vi "snake client.vi"() -> ()   [LabVIEW 2015]
uses:
  <vilib>/event_ctls.llb/eventvkey.ctl
  <vilib>/picture/picture.llb/Draw True-Color Pixmap.vi
panel:
  in  "path":path
  out "score 1":i32
  out "VKey":T1
  out "score 2":i32
  out "2D Picture":picture
  out "Numeric":i32
  out "x .and. y?":bool
  out "food x":i32
  out "food y":i32
  out "x":i32
  out "y":i32
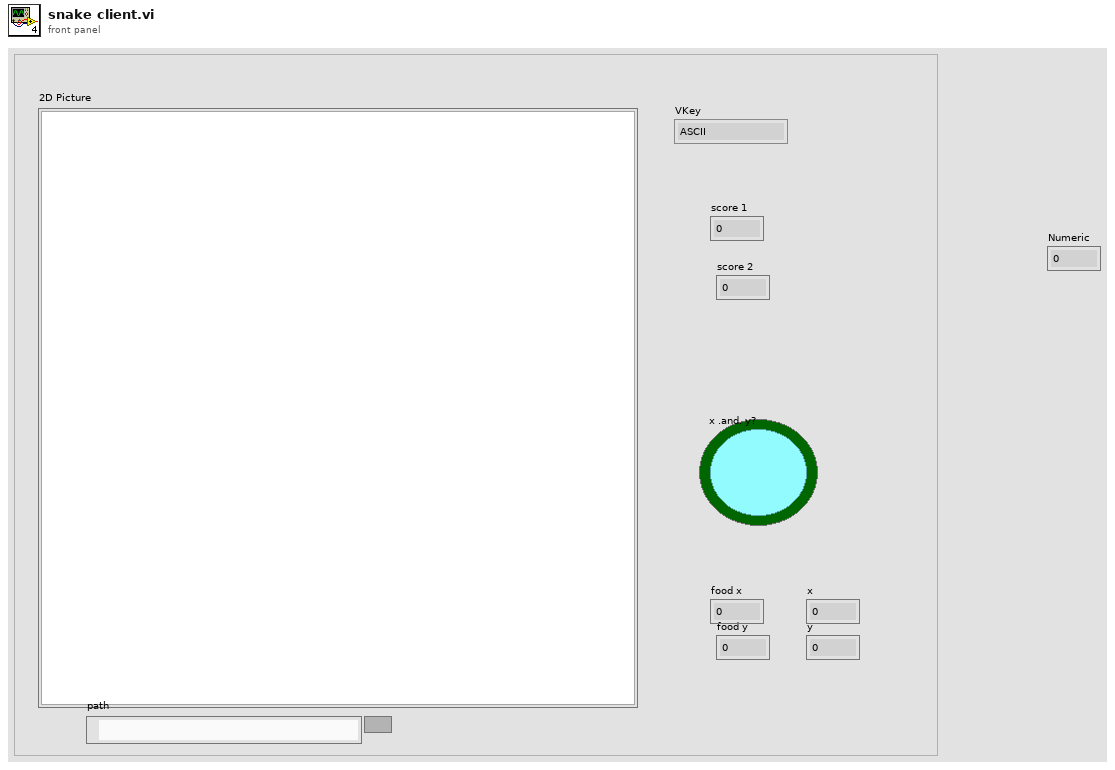
[diagram p1: front panel]
types:
  T1 = typedef "eventvkey.ctl" = enum16{"ASCII", "Enter", "Return", "Shift", "Ctrl", "Alt", "Cmd", "Opt", "Caps", "NumLock", "Clear", "Break", "Up", "Down", "Left", "Right", "Insert", "Delete", "Home", "End", "PageUp", "PageDown", "Escape", "Help", "Pause", "ScrollLock", "F1", "F2", "F3", "F4", "F5", "F6", "F7", "F8", "F9", "F10", "F11", "F12", "F13", "F14", "F15", "F16", "F17", "F18", "F19", "F20", "F21", "F22", "F23", "F24", "Play", "VolumeUp", "VolumeDown", "Mute", "Two Byte Char"}
  T2 = enum16{"Read", "Write", "ReadWrite", "BufferedRead", "BufferedReadWrite"}
  T3 = cluster{"direction":string, "snake x":i32[], "snake y":i32[]}
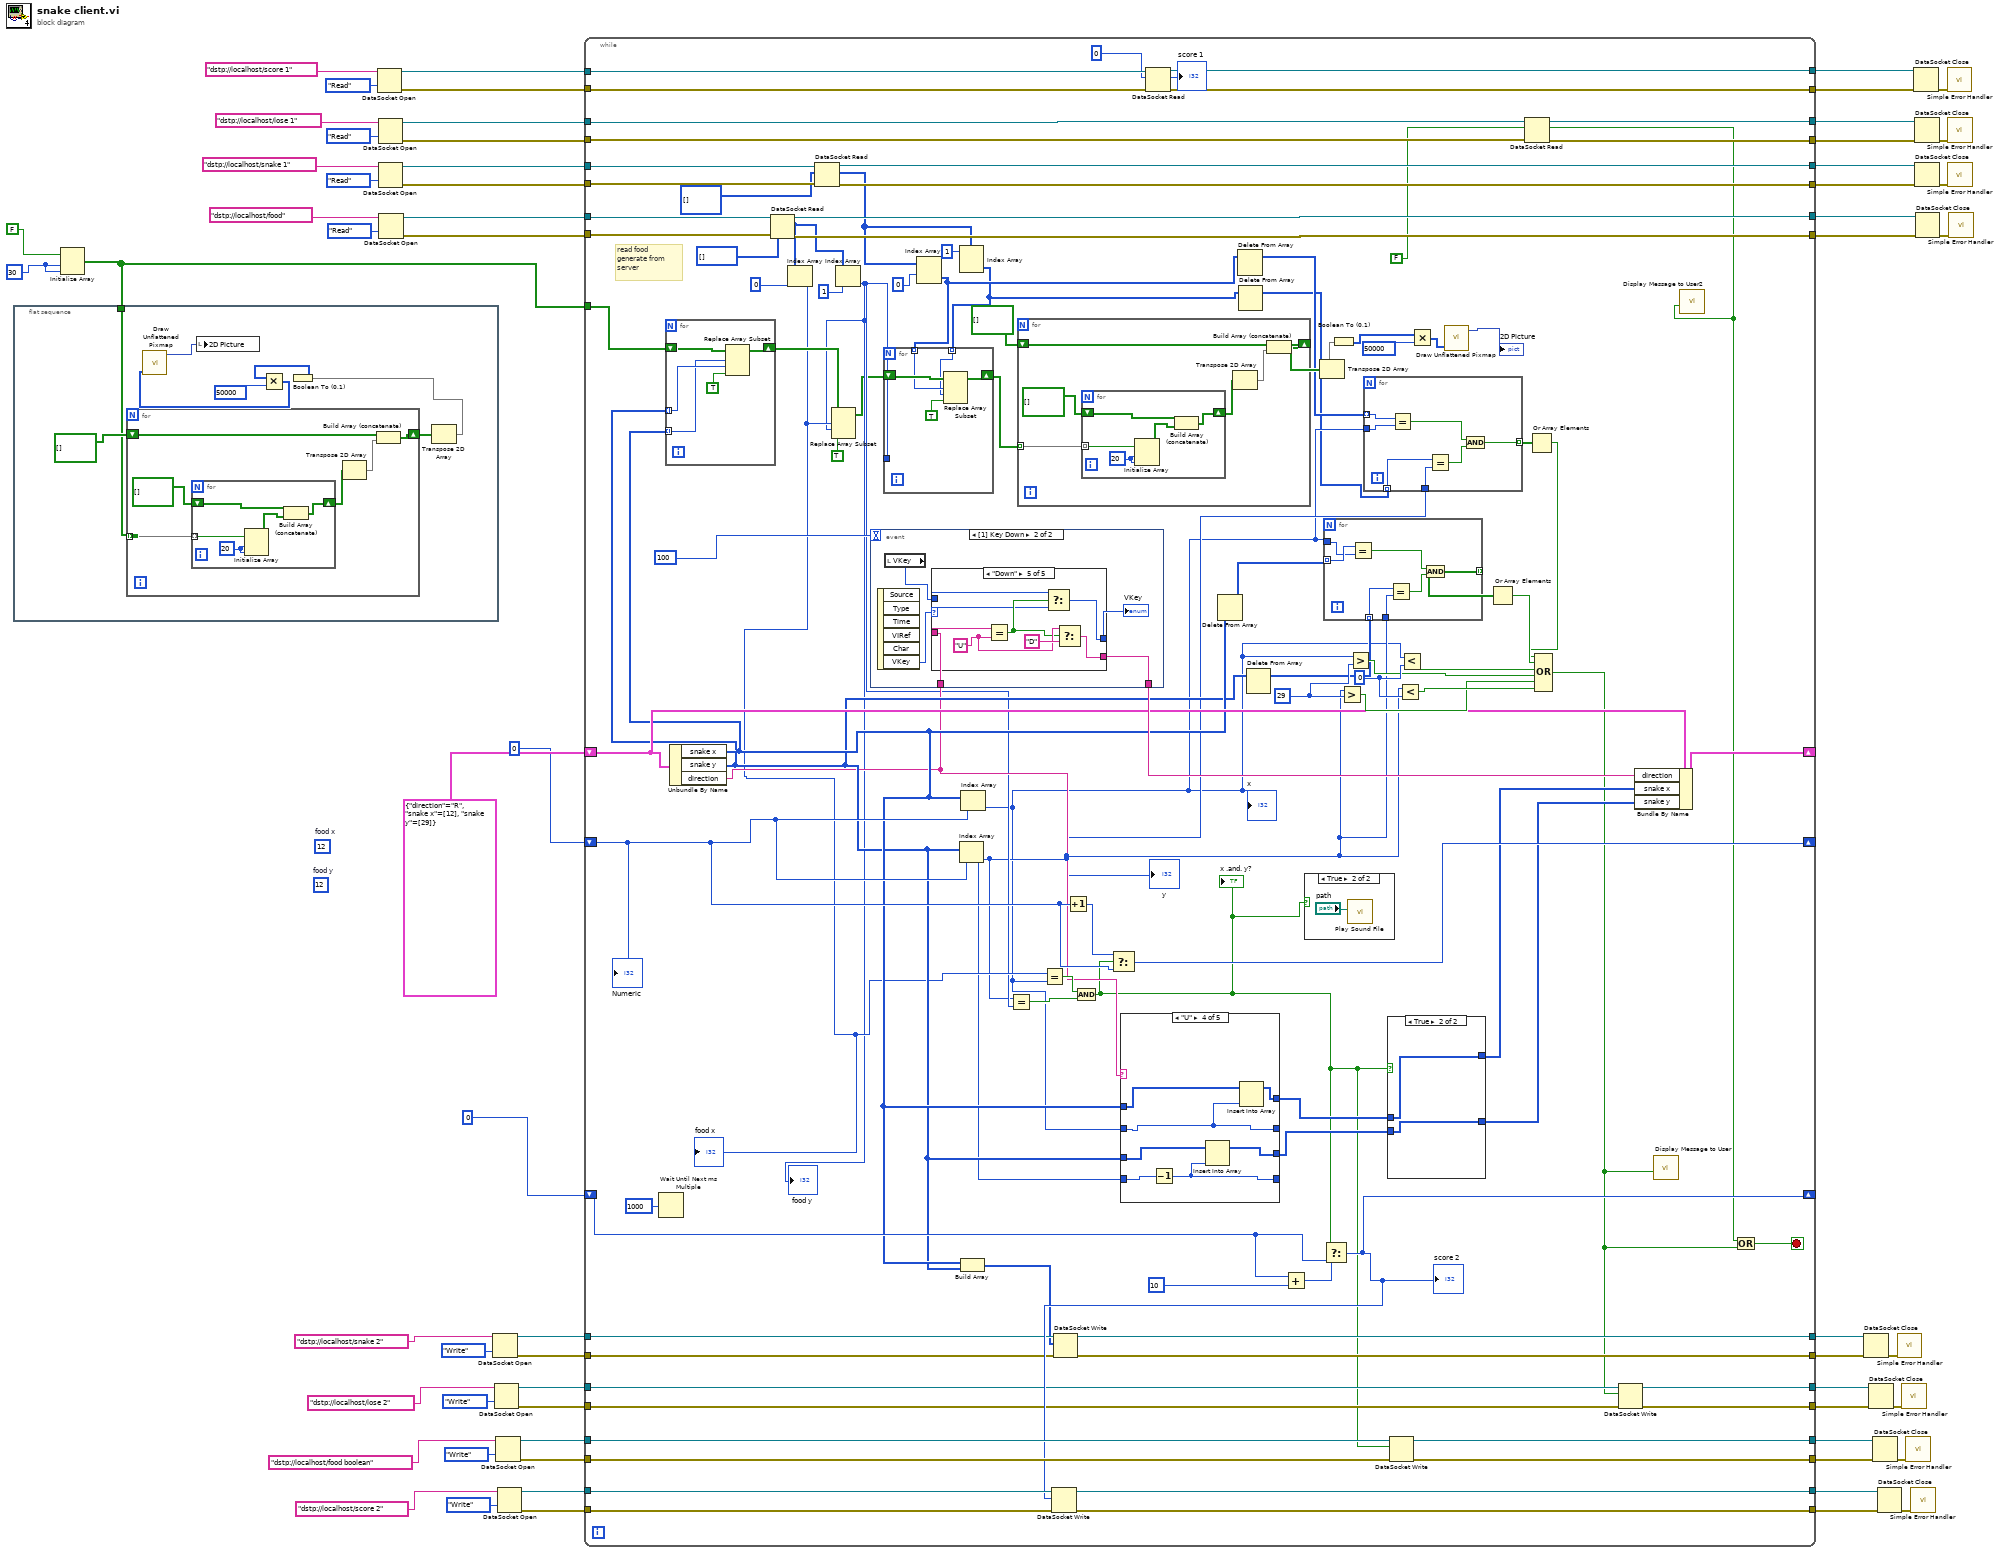
[diagram p0: block diagram]
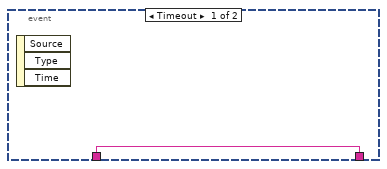
[diagram p3: hidden frame]
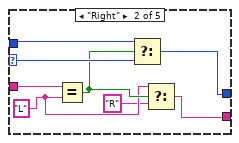
[diagram p5: hidden frame]
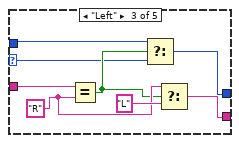
[diagram p6: hidden frame]
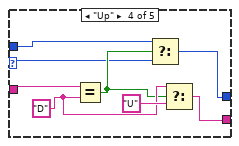
[diagram p7: hidden frame]
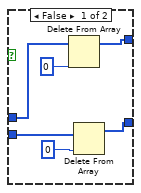
[diagram p8: hidden frame]
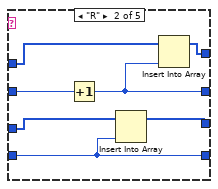
[diagram p10: hidden frame]
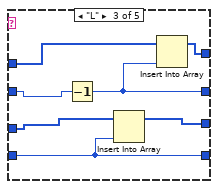
[diagram p11: hidden frame]
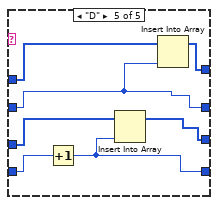
[diagram p12: hidden frame]
diagram:
  (unwired) 12  # food y
  (unwired) 12  # food x
  w59 = 30
  n1 = flat-sequence {
    tunnel: w57 -> [w63]
    frame #0 {
      n2 = for {
        tunnel: w63 -> [w76] mode=indexing
        shift-right: [w71] -> w69
        shift-left: bool[][] [] -> [w72]
        n3 = for {
          tunnel: w76 -> [w81] mode=indexing
          shift-right: [w77] -> w74
          shift-left: bool[][] [] -> [w78]
          w80 = 20
          n4 = Initialize Array(w81, w80, w80) -> (w79:bool[][])
          n5 = Build Array (concatenate)(w78, w79) -> (w77:bool[][])
        }
        n6 = Transpose 2D Array(2D array=w74) -> (transposed array=w73:bool[][])
        n7 = Build Array (concatenate)(w72, w73) -> (w71:bool[][])
      }
      n8 = Transpose 2D Array(2D array=w69) -> (transposed array=w68:bool[][])
      n9 = Boolean To (0,1)(Boolean=w68) -> (0, 1=w67:i16[][])
      n10 = Multiply(x=w67, y=50000) -> (x*y=w65:i32[][])
      n11 = call-poly <vilib>:"Draw Unflattened Pixmap.vi"("data (RGB format)"=w65) -> ("new picture"=w64:picture)  [unwired: 8 in]
      n12 = local write "2D Picture"(w64) -> ()
    }
  }
  n13 = Initialize Array(FALSE, w59, w59) -> (w57:bool[][])
  n14 = DataSocket Open(10:T2."Read" ("mode"), 11:"dstp://localhost/score 1" ("URL")) -> (0:w19:errorcluster, 3:w18:refnum<k13>)  [unwired: 2 in]
  n15 = DataSocket Open(10:T2."Read" ("mode"), 11:"dstp://localhost/lose 1" ("URL")) -> (0:w10:errorcluster, 3:w11:refnum<k13>)  [unwired: 2 in]
  n16 = DataSocket Open(10:T2."Read" ("mode"), 11:"dstp://localhost/snake 1" ("URL")) -> (0:w22:errorcluster, 3:w23:refnum<k13>)  [unwired: 2 in]
  n17 = DataSocket Open(10:T2."Read" ("mode"), 11:"dstp://localhost/food" ("URL")) -> (0:w43:errorcluster, 3:w42:refnum<k13>)  [unwired: 2 in]
  n18 = DataSocket Open(10:T2."Write" ("mode"), 11:"dstp://localhost/snake 2" ("URL")) -> (0:w34:errorcluster, 3:w33:refnum<k13>)  [unwired: 2 in]
  n19 = DataSocket Open(10:T2."Write" ("mode"), 11:"dstp://localhost/lose 2" ("URL")) -> (0:w38:errorcluster, 3:w37:refnum<k13>)  [unwired: 2 in]
  n20 = DataSocket Open(10:T2."Write" ("mode"), 11:"dstp://localhost/food boolean" ("URL")) -> (0:w55:errorcluster, 3:w56:refnum<k13>)  [unwired: 2 in]
  n21 = DataSocket Open(10:T2."Write" ("mode"), 11:"dstp://localhost/score 2" ("URL")) -> (0:w48:errorcluster, 3:w49:refnum<k13>)  [unwired: 2 in]
  n22 = while {
    shift-right: [w182] -> _
    shift-left: T3 {"direction"="R", "snake x"=[12], "snake y"=[29]} -> [w145]
    shift-right: [w178] -> _
    shift-left: 0 -> [w176]
    shift-right: [w134] -> _
    shift-left: 0 -> [w151]
    tunnel: w57 -> [w159]
    tunnel: w56 -> [w147]
    tunnel: w55 -> [w146]
    tunnel: [w144] -> w53
    tunnel: [w143] -> w52
    tunnel: w49 -> [w142]
    tunnel: w48 -> [w141]
    tunnel: [w140] -> w46
    tunnel: [w139] -> w45
    tunnel: w43 -> [w137]
    tunnel: w42 -> [w138]
    tunnel: [w136] -> w40
    tunnel: [w135] -> w39
    tunnel: w33 -> [w133]
    tunnel: w34 -> [w132]
    tunnel: w37 -> [w131]
    tunnel: w38 -> [w130]
    tunnel: [w129] -> w27
    tunnel: [w128] -> w28
    tunnel: [w127] -> w31
    tunnel: [w126] -> w32
    tunnel: w22 -> [w120]
    tunnel: w23 -> [w119]
    tunnel: [w121] -> w25
    tunnel: [w122] -> w26
    tunnel: w10 -> [w112]
    tunnel: w11 -> [w111]
    tunnel: [w113] -> w13
    tunnel: [w114] -> w14
    tunnel: w19 -> [w117]
    tunnel: w18 -> [w118]
    tunnel: [w116] -> w16
    tunnel: [w115] -> w15
    stop <- w106 stop-if-true
    w168 = 29
    w167 = 0
    # "read food\ngenerate from\nserver"
    n23 = Wait Until Next ms Multiple(millisecond multiple=u32 1000) -> ()  [unwired: 1 out]
    n24 = Unbundle By Name(w145) -> ("snake x"=w125:i32[], "snake y"=w124:i32[], "direction"=w100:string)
    n25 = for {
      tunnel: w125 -> [w207] mode=indexing
      tunnel: w124 -> [w208] mode=indexing
      shift-right: [w209] -> w158
      shift-left: w159 -> [w211]
      n26 = Replace Array Subset(array=w211, new element=TRUE, index (row)=w207, index (col)=w208) -> (w209:bool[][])
    }
    n27 = DataSocket Read(8:w137, 10:i32[] [], 11:w138) -> (0:w135:errorcluster, 2:w103:i32[], 3:w136:refnum<k13>)  [unwired: 2 in, 4 out]
    n28 = Index Array(array=w103, index=0) -> (element=w99:i32)
    "food x" <- w99
    n29 = DataSocket Read(8:w120, 10:i32[][] [], 11:w119) -> (0:w122:errorcluster, 2:w93:i32[][], 3:w121:refnum<k13>)  [unwired: 2 in, 4 out]
    n30 = Index Array(array=w103, index=1) -> (element=w97:i32)
    "food y" <- w97
    n31 = Replace Array Subset(array=w158, new element=TRUE, index (row)=w99, index (col)=w97) -> (w95:bool[][])
    n32 = event shown="[1] Key Down" {
      selector: _ -> [_ _]
      dyn-events: _ -> [_ _]
      timeout: 100 -> [_ _]
      tunnel: w100 -> [w219 w221]
      tunnel: [w219 w220] -> w174
      event Timeout {
        n33 = event-data() -> ()  [unwired: 1 in, 3 out]
      }
      event Key Down {
        n34 = event-data() -> ("VKey"=w224:T1)  [unwired: 1 in, 5 out]
        n35 = local read "VKey"() -> (w222:T1)
        n36 = case shown="\"Down\"" w224 {
          selector: w224 -> [_ w232 w238 w244 w251]
          tunnel: [w226 w231 w235 w247 w255] -> w223
          tunnel: w222 -> [w226 w233 w239 w245 w252]
          tunnel: w221 -> [w225 w234 w237 w243 w253]
          tunnel: [w225 w229 w236 w246 w254] -> w220
          frame "ASCII", Default {
          }
          frame "Right" {
            w228 = "L"
            n37 = Equal?(x=w234, y=w228) -> (x = y?=w230:bool)
            n38 = Select(t=w233, s=w230, f=w232) -> (s? t:f=w231:T1)
            n39 = Select(t=w228, s=w230, f="R") -> (s? t:f=w229:string)
          }
          frame "Left" {
            w241 = "R"
            n40 = Equal?(x=w237, y=w241) -> (x = y?=w240:bool)
            n41 = Select(t=w239, s=w240, f=w238) -> (s? t:f=w235:T1)
            n42 = Select(t=w241, s=w240, f="L") -> (s? t:f=w236:string)
          }
          frame "Up" {
            w249 = "D"
            n43 = Equal?(x=w243, y=w249) -> (x = y?=w248:bool)
            n44 = Select(t=w245, s=w248, f=w244) -> (s? t:f=w247:T1)
            n45 = Select(t=w249, s=w248, f="U") -> (s? t:f=w246:string)
          }
          frame "Down" {
            w257 = "U"
            n46 = Equal?(x=w253, y=w257) -> (x = y?=w256:bool)
            n47 = Select(t=w252, s=w256, f=w251) -> (s? t:f=w255:T1)
            n48 = Select(t=w257, s=w256, f="D") -> (s? t:f=w254:string)
          }
        }
        "VKey" <- w223
      }
    }
    n49 = Index Array(array=w93, index (row)=0) -> (element=w89:i32[])  [unwired: 1 in]
    n50 = Index Array(array=w93, index (row)=1) -> (element=w88:i32[])  [unwired: 1 in]
    n51 = for {
      tunnel: w97 -> [_]
      shift-right: [w193] -> w96
      shift-left: w95 -> [w195]
      tunnel: w89 -> [w192] mode=indexing
      tunnel: w88 -> [w191] mode=indexing
      n52 = Replace Array Subset(array=w195, new element=TRUE, index (row)=w192, index (col)=w191) -> (w193:bool[][])
    }
    n53 = Index Array(array=w124, index=w176) -> (element=w90:i32)
    "y" <- w90
    n54 = Build Array(w125, w124) -> (w123:i32[][])
    n55 = Index Array(array=w125, index=w176) -> (element=w86:i32)
    "x" <- w86
    n56 = Equal?(x=w90, y=w97) -> (x = y?=w180:bool)
    n57 = for {
      tunnel: w96 -> [w201] mode=indexing
      shift-right: [w196] -> w149
      shift-left: bool[][] [] -> [w197]
      n58 = for {
        tunnel: w201 -> [w206] mode=indexing
        shift-right: [w202] -> w199
        shift-left: bool[][] [] -> [w203]
        w205 = 20
        n59 = Initialize Array(w206, w205, w205) -> (w204:bool[][])
        n60 = Build Array (concatenate)(w203, w204) -> (w202:bool[][])
      }
      n61 = Transpose 2D Array(2D array=w199) -> (transposed array=w198:bool[][])
      n62 = Build Array (concatenate)(w197, w198) -> (w196:bool[][])
    }
    n63 = Equal?(x=w99, y=w86) -> (x = y?=w179:bool)
    n64 = DataSocket Write(8:w132, 10:w123, 11:w133) -> (0:w128:errorcluster, 3:w129:refnum<k13>)  [unwired: 1 in, 1 out]
    n65 = Increment(x=w176) -> (x+1=w177:i32)
    n66 = And(x=w179, y=w180) -> (x .and. y?=w82:bool)
    "x .and. y?" <- w82
    n67 = Select(t=w177, s=w82, f=w176) -> (s? t:f=w178:i32)
    n68 = case shown="\"U\"" w100 {
      tunnel: w125 -> [w270 w272 w283 w291 w295]
      tunnel: w124 -> [w268 w275 w281 w290 w297]
      tunnel: w86 -> [w269 w277 w282 w286 w296]
      tunnel: w90 -> [w267 w276 w280 w287 w298]
      tunnel: [w267 w276 w280 w285 w292] -> _
      tunnel: [w269 w273 w278 w286 w296] -> _
      tunnel: [w268 w274 w279 w289 w293] -> w173
      tunnel: [w270 w271 w284 w288 w294] -> w172
      frame "False", Default {
      }
      frame "R" {
        n69 = Increment(x=w277) -> (x+1=w273:i32)
        n70 = Insert Into Array(array=w275, new element=w276) -> (w274:i32[])  [unwired: 1 in]
        n71 = Insert Into Array(array=w272, new element=w273) -> (w271:i32[])  [unwired: 1 in]
      }
      frame "L" {
        n72 = Decrement(x=w282) -> (x-1=w278:i32)
        n73 = Insert Into Array(array=w281, new element=w280) -> (w279:i32[])  [unwired: 1 in]
        n74 = Insert Into Array(array=w283, new element=w278) -> (w284:i32[])  [unwired: 1 in]
      }
      frame "U" {
        n75 = Decrement(x=w287) -> (x-1=w285:i32)
        n76 = Insert Into Array(array=w290, new element=w285) -> (w289:i32[])  [unwired: 1 in]
        n77 = Insert Into Array(array=w291, new element=w286) -> (w288:i32[])  [unwired: 1 in]
      }
      frame "D" {
        n78 = Increment(x=w298) -> (x+1=w292:i32)
        n79 = Insert Into Array(array=w297, new element=w292) -> (w293:i32[])  [unwired: 1 in]
        n80 = Insert Into Array(array=w295, new element=w296) -> (w294:i32[])  [unwired: 1 in]
      }
    }
    n81 = DataSocket Read(8:w117, 10:0, 11:w118) -> (0:w115:errorcluster, 2:→"score 1":i32, 3:w116:refnum<k13>)  [unwired: 2 in, 4 out]
    n82 = Delete From Array(array=w125) -> (array with subset deleted=w91:i32[])  [unwired: 2 in, 1 out]
    n83 = Delete From Array(array=w89) -> (array with subset deleted=w87:i32[])  [unwired: 2 in, 1 out]
    n84 = Delete From Array(array=w88) -> (array with subset deleted=w85:i32[])  [unwired: 2 in, 1 out]
    n85 = Delete From Array(array=w124) -> (array with subset deleted=w161:i32[])  [unwired: 2 in, 1 out]
    n86 = Add(x=w151, y=10) -> (x+y=w160:i32)
    n87 = case shown="True" w82 {
      frame False {
      }
      frame True {
        n88 = call <vilib>:"Play Sound File.vi"("path"="path") -> ()  [unwired: 9 in, 2 out]
      }
    }
    n89 = Transpose 2D Array(2D array=w149) -> (transposed array=w148:bool[][])
    n90 = for {
      tunnel: w91 -> [w218] mode=indexing
      tunnel: w161 -> [w215] mode=indexing
      tunnel: w86 -> [w217]
      tunnel: w90 -> [w216]
      tunnel: [w212] -> w169 mode=indexing
      n91 = Equal?(x=w218, y=w217) -> (x = y?=w213:bool)
      n92 = Equal?(x=w215, y=w216) -> (x = y?=w214:bool)
      n93 = And(x=w213, y=w214) -> (x .and. y?=w212:bool)
    }
    n94 = Select(t=w160, s=w82, f=w151) -> (s? t:f=w134:i32)
    "score 2" <- w134
    n95 = DataSocket Write(8:w141, 10:w134, 11:w142) -> (0:w139:errorcluster, 3:w140:refnum<k13>)  [unwired: 1 in, 1 out]
    n96 = Boolean To (0,1)(Boolean=w148) -> (0, 1=w155:i16[][])
    n97 = Greater?(x=w90, y=w168) -> (0:w162:bool)
    n98 = Greater?(x=w86, y=w168) -> (0:w164:bool)
    n99 = for {
      tunnel: w87 -> [w190] mode=indexing
      tunnel: w85 -> [w187] mode=indexing
      tunnel: w86 -> [w189]
      tunnel: w90 -> [w188]
      tunnel: [w184] -> w84 mode=indexing
      n100 = Equal?(x=w190, y=w189) -> (x = y?=w185:bool)
      n101 = Equal?(x=w187, y=w188) -> (x = y?=w186:bool)
      n102 = And(x=w185, y=w186) -> (x .and. y?=w184:bool)
    }
    n103 = case shown="True" w82 {
      tunnel: w173 -> [w262 w265]
      tunnel: w172 -> [w261 w266]
      tunnel: [w260 w266] -> w171
      tunnel: [w259 w265] -> w170
      frame False {
        n104 = Delete From Array(array=w261, index=0) -> (array with subset deleted=w260:i32[])  [unwired: 1 in, 1 out]
        n105 = Delete From Array(array=w262, index=0) -> (array with subset deleted=w259:i32[])  [unwired: 1 in, 1 out]
      }
      frame True {
      }
    }
    n106 = DataSocket Write(8:w146, 10:w82, 11:w147) -> (0:w143:errorcluster, 3:w144:refnum<k13>)  [unwired: 1 in, 1 out]
    n107 = Less?(x=w90, y=w167) -> (x < y?=w163:bool)
    n108 = Less?(x=w86, y=w167) -> (x < y?=w165:bool)
    n109 = Multiply(x=w155, y=50000) -> (x*y=w154:i32[][])
    n110 = call-poly <vilib>:"Draw Unflattened Pixmap.vi"("data (RGB format)"=w154) -> ("new picture"=→"2D Picture":picture)  [unwired: 8 in]
    n111 = Or Array Elements(Boolean array=w169) -> (logical OR=w166:bool)
    n112 = DataSocket Read(8:w112, 10:FALSE, 11:w111) -> (0:w114:errorcluster, 2:w105:bool, 3:w113:refnum<k13>)  [unwired: 2 in, 4 out]
    n113 = Or Array Elements(Boolean array=w84) -> (logical OR=w83:bool)
    n114 = Compound Arithmetic op=OR(w83, w166, w165, w164, w162, w163) -> (w107:bool)
    n115 = DataSocket Write(8:w130, 10:w107, 11:w131) -> (0:w126:errorcluster, 3:w127:refnum<k13>)  [unwired: 1 in, 1 out]
    n116 = Bundle By Name(cluster=w145, "direction"=w174, "snake x"=w171, "snake y"=w170) -> (w182:T3)
    n117 = call "Display Message to User"("Enable"=w107) -> ()  [unwired: 9 in, 2 out]
    n118 = call "Display Message to User2"("Enable"=w105) -> ()  [unwired: 9 in, 2 out]
    n119 = Or(x=w105, y=w107) -> (x .or. y?=w106:bool)
    "Numeric" <- w176
  }
  n120 = DataSocket Close(8:w28, 11:w27) -> (0:w29:errorcluster)  [unwired: 1 in, 1 out]
  n121 = DataSocket Close(8:w32, 11:w31) -> (0:w30:errorcluster)  [unwired: 1 in, 1 out]
  n122 = DataSocket Close(8:w52, 11:w53) -> (0:w51:errorcluster)  [unwired: 1 in, 1 out]
  n123 = DataSocket Close(8:w45, 11:w46) -> (0:w47:errorcluster)  [unwired: 1 in, 1 out]
  n124 = call <vilib>:"Simple Error Handler.vi"("error in (no error)"=w29) -> ()  [unwired: 4 in, 5 out]
  n125 = call <vilib>:"Simple Error Handler.vi"("error in (no error)"=w30) -> ()  [unwired: 4 in, 5 out]
  n126 = call <vilib>:"Simple Error Handler.vi"("error in (no error)"=w51) -> ()  [unwired: 4 in, 5 out]
  n127 = call <vilib>:"Simple Error Handler.vi"("error in (no error)"=w47) -> ()  [unwired: 4 in, 5 out]
  n128 = DataSocket Close(8:w15, 11:w16) -> (0:w17:errorcluster)  [unwired: 1 in, 1 out]
  n129 = DataSocket Close(8:w14, 11:w13) -> (0:w12:errorcluster)  [unwired: 1 in, 1 out]
  n130 = DataSocket Close(8:w26, 11:w25) -> (0:w24:errorcluster)  [unwired: 1 in, 1 out]
  n131 = DataSocket Close(8:w39, 11:w40) -> (0:w41:errorcluster)  [unwired: 1 in, 1 out]
  n132 = call <vilib>:"Simple Error Handler.vi"("error in (no error)"=w17) -> ()  [unwired: 4 in, 5 out]
  n133 = call <vilib>:"Simple Error Handler.vi"("error in (no error)"=w12) -> ()  [unwired: 4 in, 5 out]
  n134 = call <vilib>:"Simple Error Handler.vi"("error in (no error)"=w24) -> ()  [unwired: 4 in, 5 out]
  n135 = call <vilib>:"Simple Error Handler.vi"("error in (no error)"=w41) -> ()  [unwired: 4 in, 5 out]
